vi "A170316-11-Main-large.vi"() -> ()   [LabVIEW 2020]
uses:
  System.Windows.Forms
  Global_Variable/Global.vi
  Database/Global1.vi
  <userlib>/_MGI/Menu Building/MenuItemStatusChange/MGI_MenuItemStatusChange.lvclass
  Libraries/S7/S7.lvlib
panel:
  out "PLC":bool
  out "传感器值":sgl format="%#_5gN"
  out "前序状态字":string
  out "前序状态":bool
  in  "打印条码":bool caption="布尔"
  out "结果显示":string
  in  "质量报警":bool caption="布尔"
  in  "设备缺料":bool caption="布尔"
  in  "设备故障":bool caption="布尔"
  in  "设备离线":bool caption="布尔"
  in  "设备正常":bool caption="布尔"
  in  "菜单":refnum<k24>(container)
  out "检测结果":bool
  in  "批次信息":string[][](table)
  out "提示信息":string
  out "错误":bool
  out "时间字符串":string
  out "日期字符串":string
  out "自动":bool
  out "userStatus":string caption="用户状态"
  out "userName":string caption="用户名"
  out "合格数量":u32
  out "生产数量":u32
  out "追溯码":string
  out "connectionMode":string caption="联机类型"
  out "产品型号":string
  in  "更换产品":refnum<vi>
  # "中间轴装配"
  # "工艺流程"
  # "检测结果："
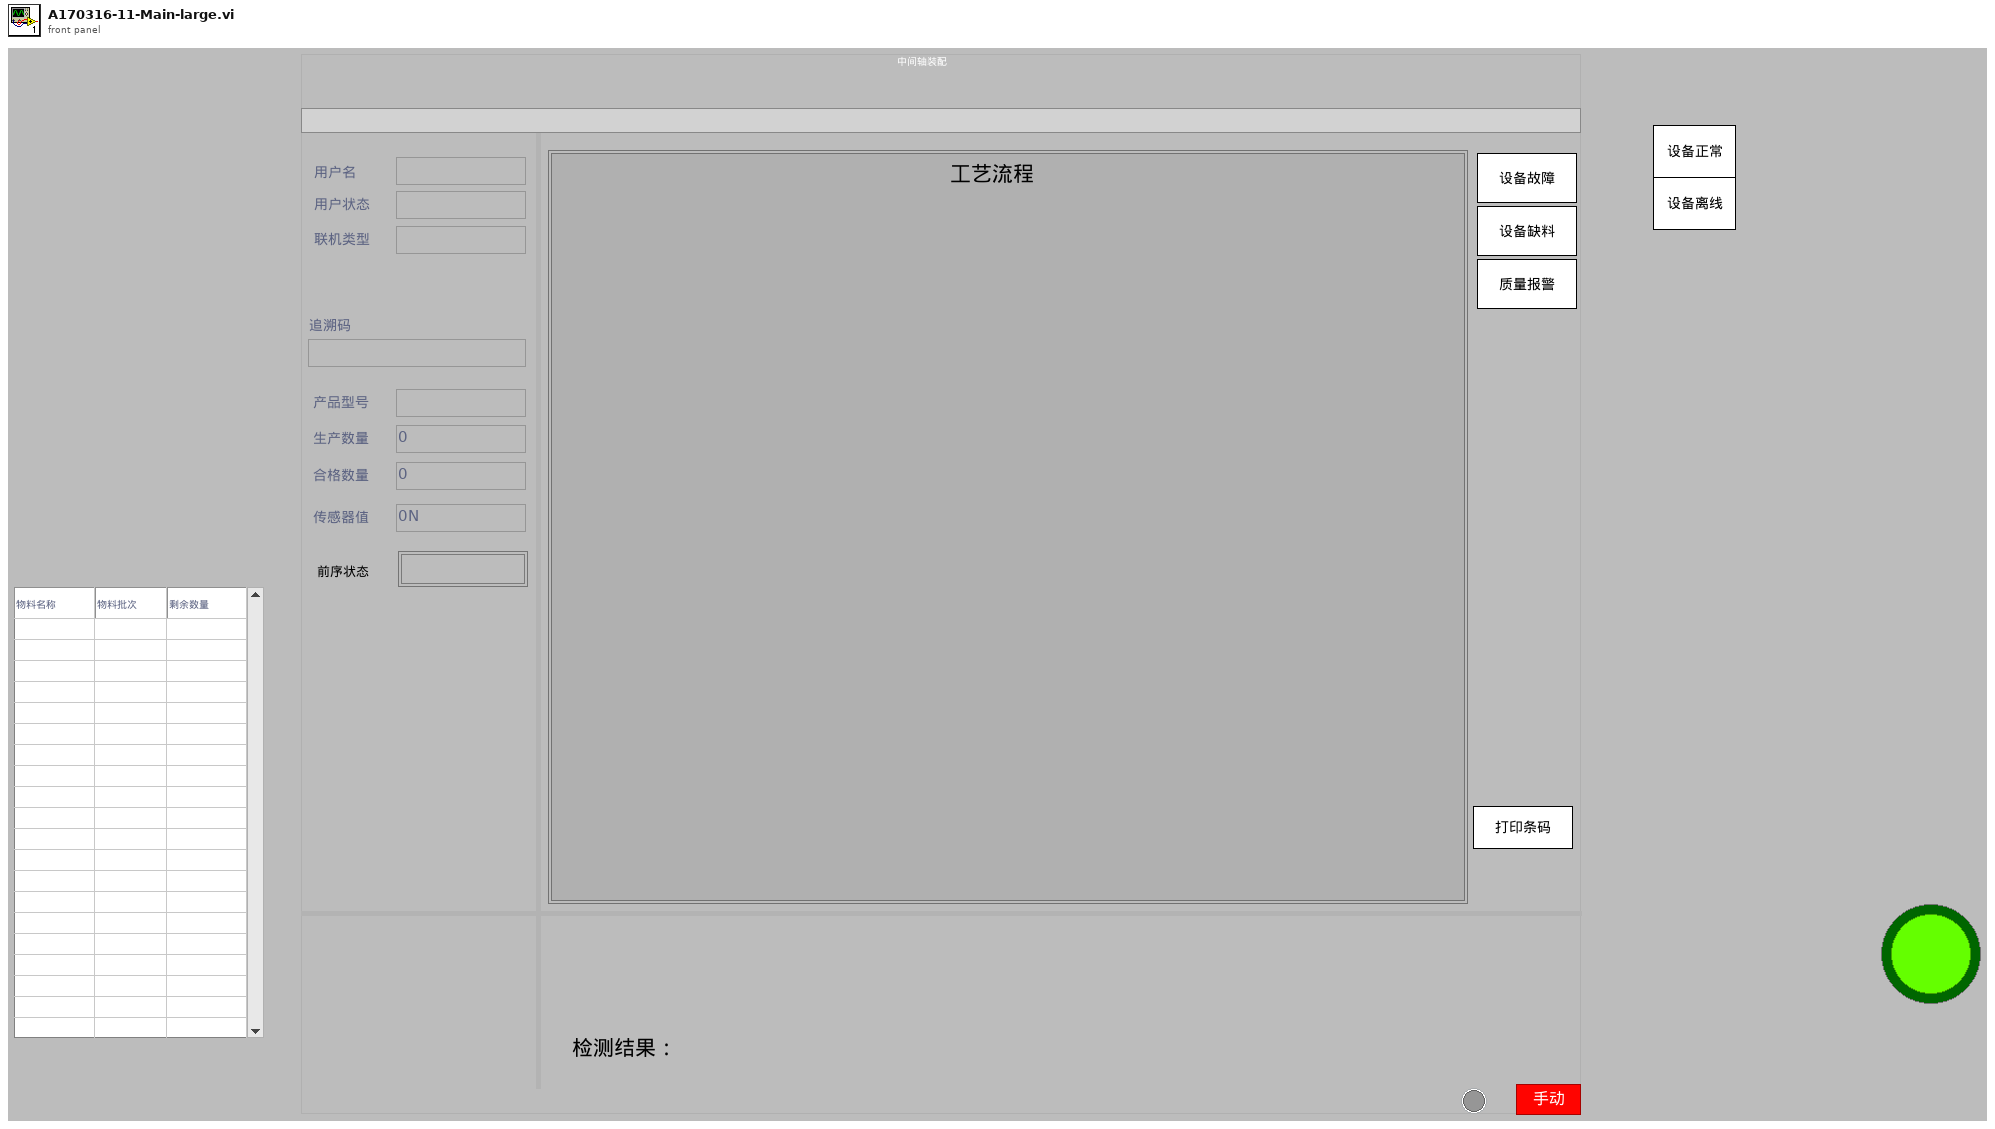
[diagram p1: front panel]
types:
  T1 = typedef "S7.lvlib/Broadcast Events--cluster.ctl" = cluster{"Module Did Init":refnum<user-event>, "Status Updated":refnum<user-event>, "Error Reported":refnum<user-event>, "Module Did Stop":refnum<user-event>, "Update Module Execution Status":refnum<user-event>}
  T2 = enum32{"Invalid", "Standard", "Closed", "Hidden", "Minimized", "Maximized"}
  T3 = enum32{"invalid app kind", "Development System", "Run Time System", "Student Edition", "Embedded LabVIEW", "Evaluation", "Custom"}
  T4 = typedef "S7.lvlib/Read_Data (Reply Payload)--cluster.ctl" = cluster{"读取成功":bool, "数据":u32[], "Read_Data_error":errorcluster}
  T5 = cluster{"Core":cluster{"Current VI Reference":refnum<vi>, "Close Panel on Exit?":bool}, "Your Boolean data":bool, "Your string data":string}
  T6 = cluster{"Current VI Reference":refnum<vi>, "Close Panel on Exit?":bool}
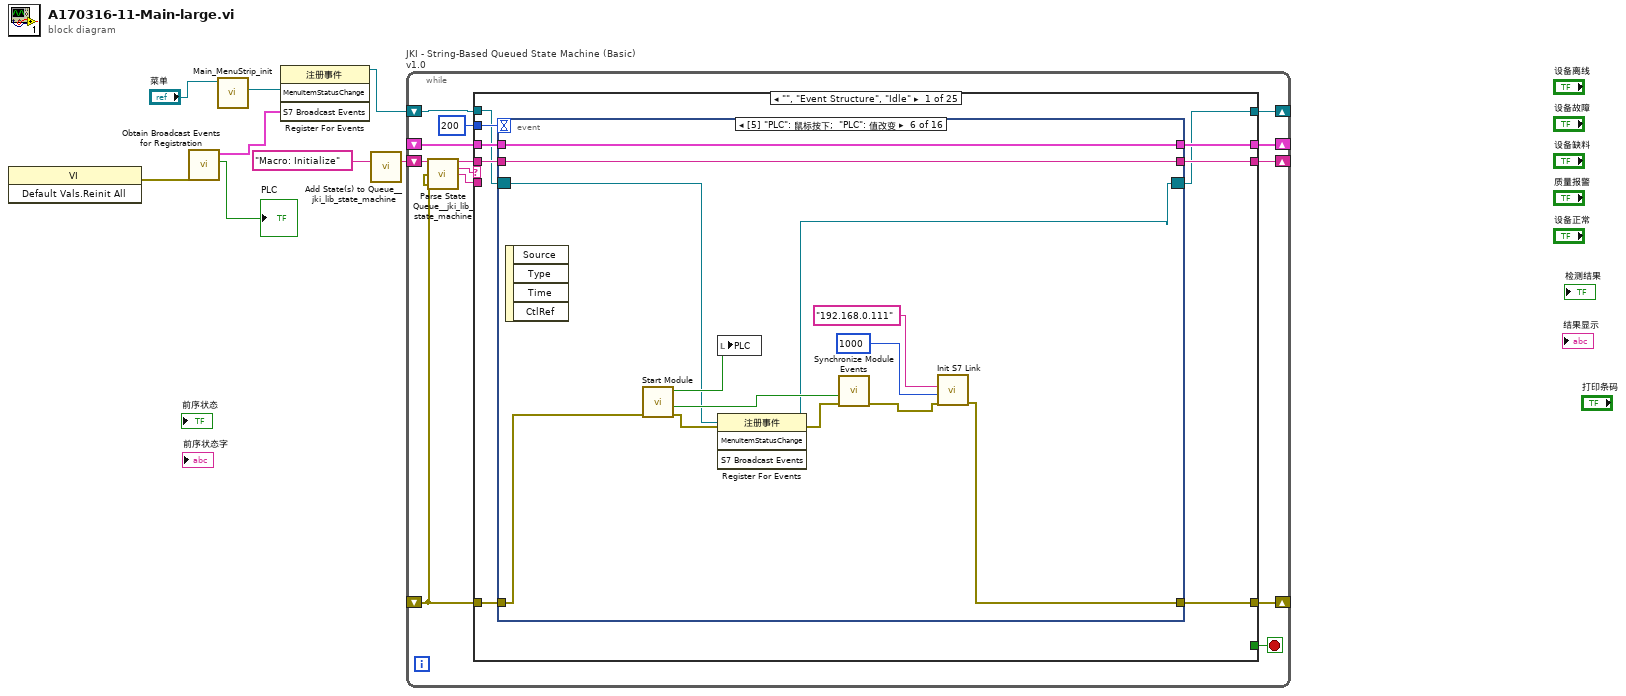
[diagram p0: block diagram]
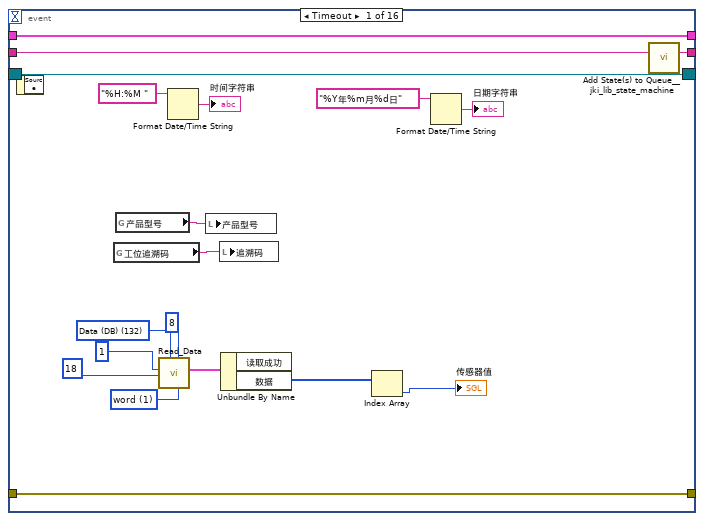
[diagram p2: hidden frame]
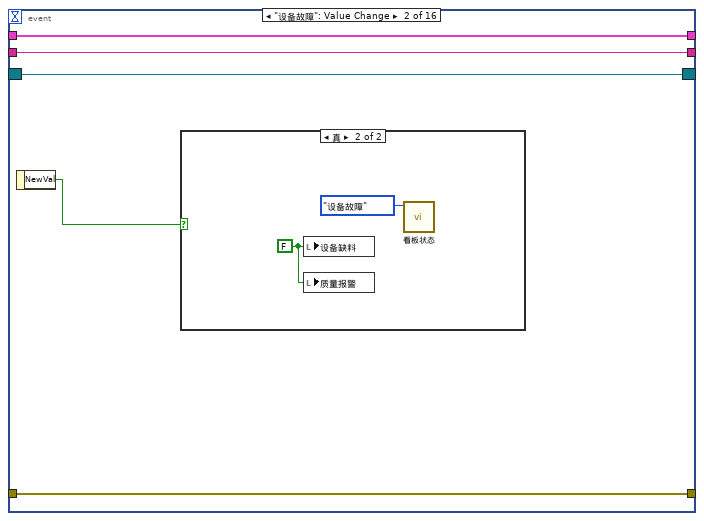
[diagram p3: hidden frame]
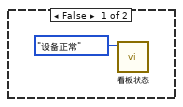
[diagram p4: hidden frame]
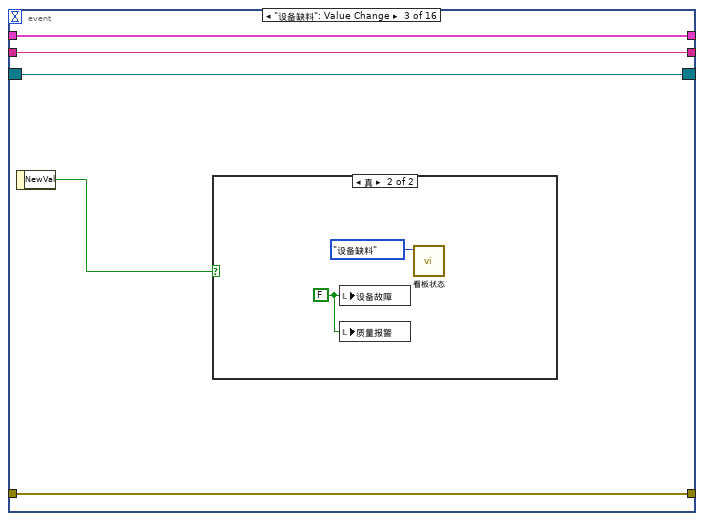
[diagram p5: hidden frame]
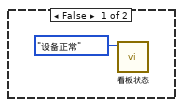
[diagram p6: hidden frame]
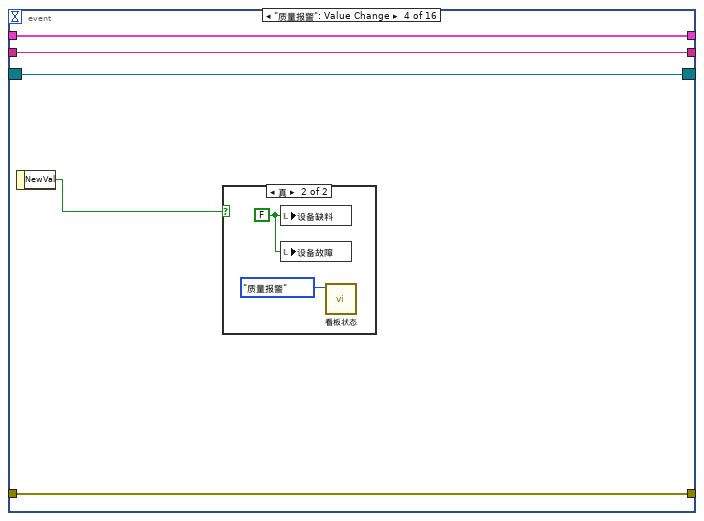
[diagram p7: hidden frame]
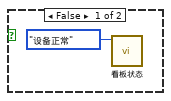
[diagram p8: hidden frame]
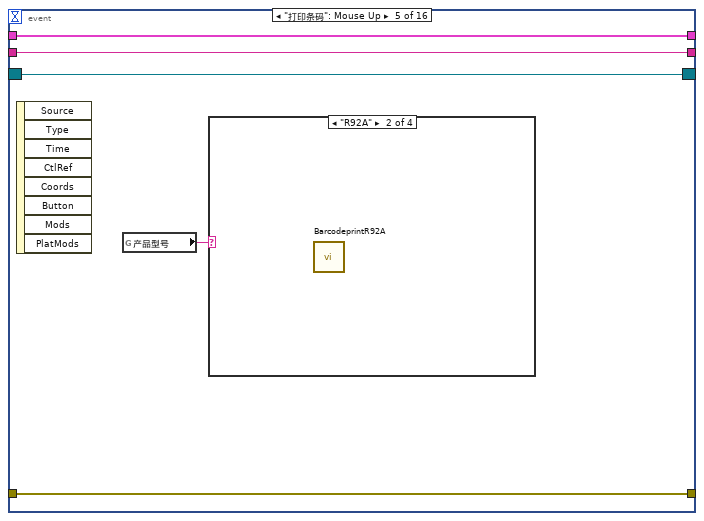
[diagram p9: hidden frame]
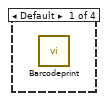
[diagram p10: hidden frame]
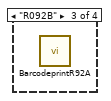
[diagram p11: hidden frame]
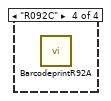
[diagram p12: hidden frame]
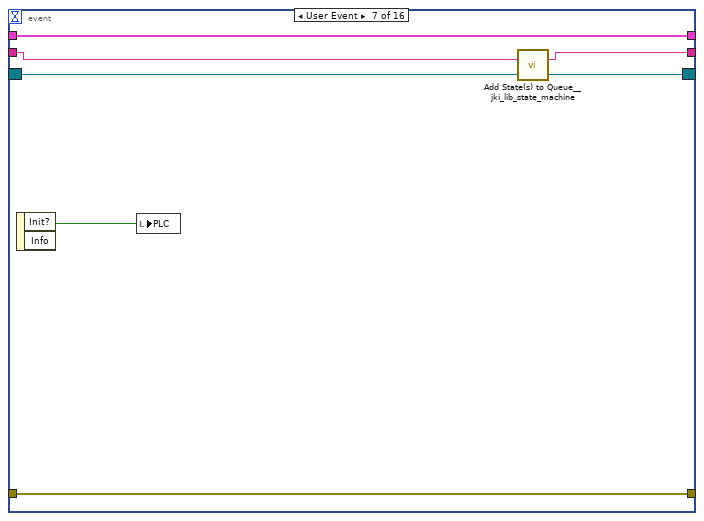
[diagram p13: hidden frame]
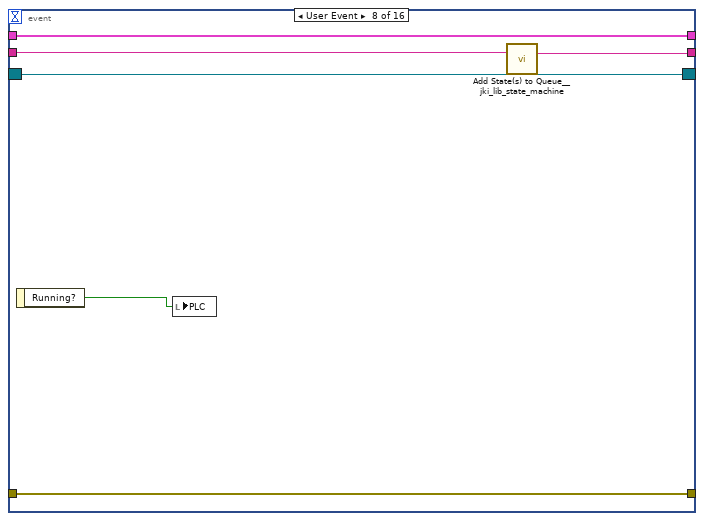
[diagram p14: hidden frame]
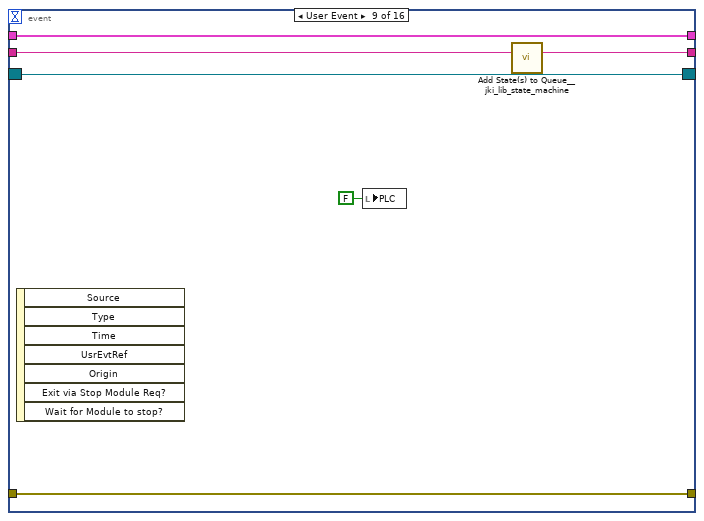
[diagram p15: hidden frame]
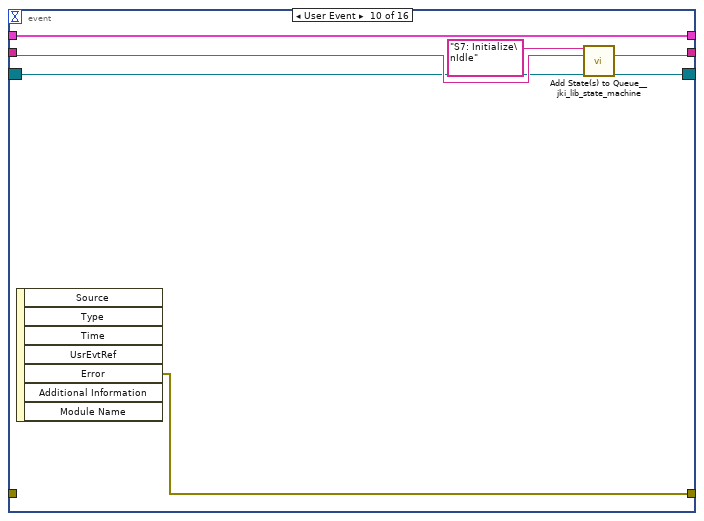
[diagram p16: hidden frame]
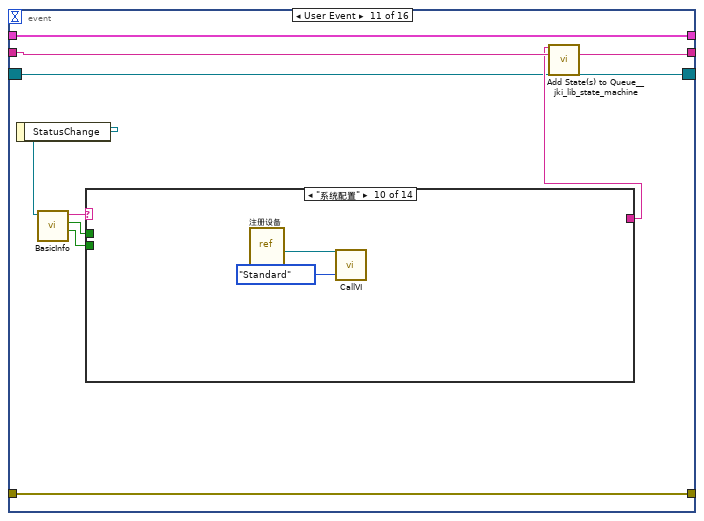
[diagram p17: hidden frame]
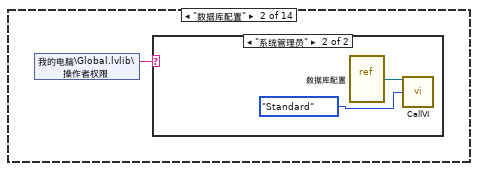
[diagram p19: hidden frame]
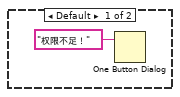
[diagram p20: hidden frame]
diagram:
  n1 = invoke class="VI" method="Default Vals.Reinit All"() -> (error out=w4:errorcluster)  [unwired: 3 in, 2 out]
  n2 = call "Obtain Broadcast Events for Registration.vi"("error in (no error)"=w4) -> ("Already running?"=→"PLC":bool, "S7 Broadcast Events"=w3:T1)  [unwired: 8 in, 1 out]
  n3 = call "Main_MenuStrip_init.vi"("MenuStrip"="菜单") -> ("MenuItemStatusChange"=w5:refnum<user-event>)  [unwired: 9 in, 1 out]
  n4 = register-events(w5, w3) -> (reference out=w2:refnum<event-registration>)  [unwired: 2 in, 1 out]
  n5 = call <vilib>:"Add State(s) to Queue__jki_lib_state_machine.vi"("State(s) in (\"\")"="Macro: Initialize") -> ("States Out"=w8:string)  [unwired: 14 in]
  n6 = while "JKI - String-Based Queued State Machine (Basic) v1.0" {
    shift-right: [w14] -> _
    shift-left: _ -> [w13]
    shift-right: [w17] -> _
    shift-left: _ -> [w11]
    shift-right: [w16] -> _
    shift-left: w8 -> [w18]
    shift-right: [w10] -> _
    shift-left: w2 -> [w9]
    stop <- w15 stop-if-true
    n7 = call <vilib>:"Parse State Queue__jki_lib_state_machine.vi"("State Queue"=w18, "Error In (no error)"=w11) -> ("Remaining States"=w20:string, "Current State"=w21:string, "Arguments"=w19:string)  [unwired: 11 in]
    n8 = case shown="\"\", \"Event Structure\", \"Idle\"" w21 {
      selector: w21 -> [_ _ w261 _ _ _ _ _ _ _ _ _ _ _ _ _ _ _ _ _ _ _ _ _ _]
      tunnel: w20 -> [w30 w259 w265 w283 w289 w294 w298 w305 w311 w315 w316 w323 w327 w331 w335 w347 w351 w390 w401 w427 w432 w445 w449 w453 w457]
      tunnel: w19 -> [_ _ _ _ _ _ _ _ _ _ _ _ _ _ _ _ _ w385 w395 _ _ _ _ _ _]
      tunnel: w13 -> [w28 w256 w263 w274 w286 w292 w295 _ w306 w312 w318 w320 w324 w328 w332 w345 w349 w388 w397 w424 w429 w442 w446 w450 w454]
      tunnel: [w27 w257 w267 w280 errorcluster {"status"=FALSE, "code"=0, "source"=""} ("error out") w291 w296 w302 w307 w313 w319 w321 w325 w329 w333 w342 w348 w386 w398 w425 w430 w443 w447 w451 w455] -> w17
      tunnel: w11 -> [w26 w257 w266 w280 w285 w291 w296 w302 w308 w313 w319 w321 w325 w329 w333 w337 w348 w387 w399 w425 w430 w443 w447 w451 w455]
      tunnel: [w29 w258 w264 w282 w288 w293 w297 w304 w310 w314 w316 w322 w326 w330 w334 w346 w350 w389 w400 w426 w431 w444 w448 w452 w456] -> w16
      tunnel: [_ _ _ _ _ TRUE _ _ _ _ _ _ _ _ _ _ _ _ _ _ _ _ _ _ _] -> w15
      tunnel: [w25 w256 w263 w281 w286 w292 w295 w303 w306 w312 w318 w320 w324 w328 w332 w345 w349 w388 w397 w424 w429 w442 w446 w450 w454] -> w14
      tunnel: 200 ("Timeout") -> [w24 _ _ _ _ _ _ _ _ _ _ _ _ _ _ _ _ _ _ _ _ _ _ _ _]
      tunnel: w9 -> [w23 _ w260 _ _ _ _ _ _ _ _ _ _ _ _ _ _ _ _ _ _ _ _ _ _]
      tunnel: [w22 _ w260 _ _ _ _ _ _ _ _ _ _ _ _ _ _ _ _ _ _ _ _ _ _] -> w10
      frame "", "Event Structure", "Idle" {
        n9 = event shown="[5] \"PLC\": 鼠标按下;  \"PLC\": 值改变" {
          selector: w23 -> [w31 w50 w58 w66 w74 w88 w92 w98 w104 w110 w116 w168 w218 w225 w241 w249]
          dyn-events: [w31 w50 w58 w66 w74 w87 w92 w98 w104 w110 w116 w168 w218 w225 w241 w249] -> w22
          timeout: w24 -> [_ _ _ _ _ _ _ _ _ _ _ _ _ _ _ _]
          tunnel: w30 -> [w49 w53 w61 w69 w76 w85 w95 w102 w107 w111 w120 w171 w222 w229 w248 w252]
          tunnel: [w48 w53 w61 w69 w76 w85 w94 w101 w108 w112 w119 w169 w223 w229 w247 w253] -> w29
          tunnel: w28 -> [w46 w54 w62 w70 w77 w86 w96 w100 w106 w114 w121 w170 w224 w230 w245 w255]
          tunnel: [w47 w52 w60 w68 w75 w79 w93 w99 w105 w115 w117 w172 w221 w228 w246 w254] -> w27
          tunnel: w26 -> [w47 w52 w60 w68 w75 w90 w93 w99 w105 _ w117 w172 w221 w228 w246 w254]
          tunnel: [w46 w54 w62 w70 w77 w86 w96 w100 w106 w114 w121 w170 w224 w230 w245 w255] -> w25
          event Timeout {
            w32 = u16 1 items=["byte", "word", "Dword"] ("数据类型")
            w38 = u8 132 items=["I/O (P)"=128, "Input (I)"=129, "Output (Q)"=130, "Bit Memory (M)"=131, "Data (DB)"=132, "Instance Data (DI)"=133, "Local Data (L)"=134, "Predecessor Local Data (VL)"=135] ("寄存器类型")
            n10 = event-data() -> ()  [unwired: 1 in, 1 out]
            n11 = global read "Global1.vi" "工位追溯码"() -> (w40:string)
            n12 = global read "Global.vi" "产品型号"() -> (w41:string)
            n13 = call "Read_Data.vi"("数据类型"=w32, "读取长度"=u16 8, "寄存器类型"=w38, "起始地址"=u32 18, "DB #"=u16 1) -> ("Reply Payload"=w35:T4)  [unwired: 4 in, 2 out]
            n14 = Format Date/Time String(time format string (%c)="%H:%M ") -> (date/time string=→"时间字符串":string)  [unwired: 2 in]
            n15 = local write "产品型号"(w41) -> ()
            n16 = local write "追溯码"(w40) -> ()
            n17 = Unbundle By Name(w35) -> ("数据"=w34:u32[])  [unwired: 1 out]
            n18 = Index Array(array=w34) -> (element=→"传感器值":u32)  [unwired: 1 in]
            n19 = Format Date/Time String(time format string (%c)="%Y年%m月%d日") -> (date/time string=→"日期字符串":string)  [unwired: 2 in]
            n20 = call <vilib>:"Add State(s) to Queue__jki_lib_state_machine.vi"("State(s) in (\"\")"=w49) -> ("States Out"=w48:string)  [unwired: 14 in]
          }
          event "设备故障": Value Change {
            n21 = event-data() -> ("NewVal"=w51:bool)  [unwired: 1 in]
            n22 = case shown="真" w51 {
              frame False {
                n23 = call "看板状态.vi"("设备状态"=enum16{"设备离线", "设备正常", "设备缺料", "设备故障", "质量报警"}."设备正常") -> ()  [unwired: 10 in, 1 out]
              }
              frame True {
                w56 = FALSE ("质量报警")
                n24 = local write "设备缺料"(w56) -> ()
                n25 = local write "质量报警"(w56) -> ()
                n26 = call "看板状态.vi"("设备状态"=enum16{"设备离线", "设备正常", "设备缺料", "设备故障", "质量报警"}."设备故障") -> ()  [unwired: 10 in, 1 out]
              }
            }
          }
          event "设备缺料": Value Change {
            n27 = event-data() -> ("NewVal"=w59:bool)  [unwired: 1 in]
            n28 = case shown="真" w59 {
              frame False {
                n29 = call "看板状态.vi"("设备状态"=enum16{"设备离线", "设备正常", "设备缺料", "设备故障", "质量报警"}."设备正常") -> ()  [unwired: 10 in, 1 out]
              }
              frame True {
                w64 = FALSE ("质量报警")
                n30 = local write "设备故障"(w64) -> ()
                n31 = local write "质量报警"(w64) -> ()
                n32 = call "看板状态.vi"("设备状态"=enum16{"设备离线", "设备正常", "设备缺料", "设备故障", "质量报警"}."设备缺料") -> ()  [unwired: 10 in, 1 out]
              }
            }
          }
          event "质量报警": Value Change {
            n33 = event-data() -> ("NewVal"=w67:bool)  [unwired: 1 in]
            n34 = case shown="真" w67 {
              frame False {
                n35 = call "看板状态.vi"("设备状态"=enum16{"设备离线", "设备正常", "设备缺料", "设备故障", "质量报警"}."设备正常") -> ()  [unwired: 10 in, 1 out]
              }
              frame True {
                w72 = FALSE ("质量报警")
                n36 = local write "设备缺料"(w72) -> ()
                n37 = local write "设备故障"(w72) -> ()
                n38 = call "看板状态.vi"("设备状态"=enum16{"设备离线", "设备正常", "设备缺料", "设备故障", "质量报警"}."质量报警") -> ()  [unwired: 10 in, 1 out]
              }
            }
          }
          event "打印条码": Mouse Up {
            n39 = event-data() -> ()  [unwired: 1 in, 8 out]
            n40 = global read "Global.vi" "产品型号"() -> (w78:string)
            n41 = case shown="\"R92A\"" w78 {
              frame Default {
                n42 = call "Barcodeprint.vi"() -> ()  [unwired: 12 in]
              }
              frame "R92A" {
                n43 = call "BarcodeprintR92A.vi"() -> ()  [unwired: 12 in]
              }
              frame "R092B" {
                n44 = call "BarcodeprintR92A.vi"() -> ()  [unwired: 12 in]
              }
              frame "R092C" {
                n45 = call "BarcodeprintR92A.vi"() -> ()  [unwired: 12 in]
              }
            }
          }
          event "PLC": Mouse Down; "PLC": Value Change {
            n46 = event-data() -> ()  [unwired: 1 in, 4 out]
            n47 = call "Start Module.vi"("error in (no error)"=w90) -> ("error out"=w80:errorcluster, "Wait for Event Sync?"=w89:bool, "Module Was Already Running?"=w91:bool)  [unwired: 7 in, 1 out]
            n48 = local write "PLC"(w91) -> ()
            n49 = register-events(reference=w88, error in=w80) -> (reference out=w87:refnum<event-registration>, error out=w81:errorcluster)  [unwired: 2 in]
            n50 = call "Synchronize Module Events.vi"("error in (no error)"=w81, "Wait for Event Sync?"=w89) -> ("error out"=w82:errorcluster)  [unwired: 9 in]
            n51 = call "Init S7 Link.vi"("error in (no error)"=w82, "超时"=1000, "IP"="192.168.0.111" ("Origin")) -> ("error out"=w79:errorcluster)  [unwired: 8 in]
          }
          event User Event {
            n52 = event-data() -> ("Init?"=w97:bool)  [unwired: 1 in, 1 out]
            n53 = local write "PLC"(w97) -> ()
            n54 = call <vilib>:"Add State(s) to Queue__jki_lib_state_machine.vi"("State(s) in (\"\")"=w95) -> ("States Out"=w94:string)  [unwired: 14 in]
          }
          event User Event {
            n55 = event-data() -> ("Running?"=w103:bool)  [unwired: 1 in]
            n56 = local write "PLC"(w103) -> ()
            n57 = call <vilib>:"Add State(s) to Queue__jki_lib_state_machine.vi"("State(s) in (\"\")"=w102) -> ("States Out"=w101:string)  [unwired: 14 in]
          }
          event User Event {
            n58 = event-data() -> ()  [unwired: 1 in, 7 out]
            n59 = local write "PLC"(FALSE ("PLC")) -> ()
            n60 = call <vilib>:"Add State(s) to Queue__jki_lib_state_machine.vi"("State(s) in (\"\")"=w107) -> ("States Out"=w108:string)  [unwired: 14 in]
          }
          event User Event {
            n61 = event-data() -> ("Error"=w115:errorcluster)  [unwired: 1 in, 6 out]
            n62 = call <vilib>:"Add State(s) to Queue__jki_lib_state_machine.vi"("State(s) in Front (\"\")"="S7: Initialize\nIdle" ("State(s) in Front (\"\")"), "State(s) in (\"\")"=w111) -> ("States Out"=w112:string)  [unwired: 13 in]
          }
          event User Event {
            n63 = event-data() -> ("StatusChange"=w122:refnum<class "MGI_MenuItemStatusChange.lvclass">)  [unwired: 1 in]
            n64 = call <userlib>:"BasicInfo.vi"("MGI_MenuItemStatusChange in"=w122) -> ("Enabled?"=w125:bool, "Checked?"=w124:bool, "Tag"=w123:string)  [unwired: 7 in, 1 out]
            n65 = case shown="\"系统配置\"" w123 {
              tunnel: w124 -> [_ _ _ _ _ _ _ _ _ _ _ _ _ _]
              tunnel: w125 -> [_ _ _ _ _ _ _ _ _ _ _ _ _ _]
              tunnel: [_ _ "Macro: Exit" _ _ _ _ _ _ _ _ _ _ _] -> w118
              frame Default {
              }
              frame "数据库配置" {
                n66 = shared-variable "我的电脑\\Global.lvlib\\操作者权限"() -> (w126:string)  [unwired: 1 in, 1 out]
                n67 = case shown="\"系统管理员\"" w126 {
                  frame Default {
                    n68 = One Button Dialog(message="权限不足！" ("消息")) -> ()  [unwired: 1 in, 1 out]
                  }
                  frame "系统管理员" {
                    n69 = vi-ref "数据库配置.vi"() -> (w129:refnum<vi>)
                    n70 = call "CallVI.vi"("VI引用"=w129, "状态"=T2."Standard") -> ()  [unwired: 11 in, 3 out]
                  }
                }
              }
              frame "退出" {
              }
              frame "手动控制" {
                n71 = shared-variable "我的电脑\\Global.lvlib\\操作者权限"() -> (w131:string)  [unwired: 1 in, 1 out]
                n72 = case shown="\"班组长\", \"系统管理员\"" w131 {
                  frame Default {
                    n73 = One Button Dialog(message="权限不足！" ("消息")) -> ()  [unwired: 1 in, 1 out]
                  }
                  frame "班组长", "系统管理员" {
                    n74 = vi-ref "A170316-11_IO.vi"() -> (w134:refnum<vi>)
                    n75 = call "CallVI.vi"("VI引用"=w134, "状态"=T2."Standard") -> ()  [unwired: 11 in, 3 out]
                  }
                }
              }
              frame "产品管理" {
                n76 = vi-ref "A170316-11_config.vi"() -> (w136:refnum<vi>)
                n77 = call "CallVI.vi"("VI引用"=w136, "状态"=T2."Standard") -> ()  [unwired: 11 in, 3 out]
              }
              frame "用户管理" {
                n78 = shared-variable "我的电脑\\Global.lvlib\\操作者权限"() -> (w137:string)  [unwired: 1 in, 1 out]
                n79 = case shown="\"系统管理员\"" w137 {
                  frame Default {
                    n80 = One Button Dialog(message="权限不足！" ("消息")) -> ()  [unwired: 1 in, 1 out]
                  }
                  frame "系统管理员" {
                    n81 = vi-ref "User_manager.vi"() -> (w140:refnum<vi>)
                    n82 = call "CallVI.vi"("VI引用"=w140, "状态"=T2."Standard") -> ()  [unwired: 11 in, 3 out]
                  }
                }
              }
              frame "编码规则" {
                n83 = shared-variable "我的电脑\\Global.lvlib\\操作者权限"() -> (w141:string)  [unwired: 1 in, 1 out]
                n84 = case shown="\"班组长\", \"工艺管理员\", \"系统管理员\"" w141 {
                  frame Default {
                    n85 = One Button Dialog(message="权限不足！" ("消息")) -> ()  [unwired: 1 in, 1 out]
                  }
                  frame "班组长", "工艺管理员", "系统管理员" {
                    n86 = vi-ref "编码规则设置.vi"() -> (w144:refnum<vi>)
                    n87 = call "CallVI.vi"("VI引用"=w144, "状态"=T2."Standard") -> ()  [unwired: 11 in, 3 out]
                  }
                }
              }
              frame "易损件管理" {
                n88 = vi-ref "易损件管理.vi"() -> (w146:refnum<vi>)
                n89 = call "CallVI.vi"("VI引用"=w146, "状态"=T2."Standard") -> ()  [unwired: 11 in, 3 out]
              }
              frame "物料批次管理" {
                n90 = vi-ref "批次管理.vi"() -> (w148:refnum<vi>)
                n91 = call "CallVI.vi"("VI引用"=w148, "状态"=T2."Standard") -> ()  [unwired: 11 in, 3 out]
              }
              frame "系统配置" {
                n92 = vi-ref "注册设备.vi"() -> (w150:refnum<vi>)
                n93 = call "CallVI.vi"("VI引用"=w150, "状态"=T2."Standard") -> ()  [unwired: 11 in, 3 out]
              }
              frame "报表" {
                n94 = call "文件对话框2"("start path"=path "D:/report", "prompt"="打开报表", "pattern (all files)"="*.doc;*.docx", "pattern label"="Word 文档") -> ("selected path"=w151:path, "error out"=w152:errorcluster)  [unwired: 8 in, 2 out]
                n95 = case shown="无错误" w152 {
                  selector: w152 -> [w158 w160]
                  tunnel: w151 -> [w159 _]
                  frame No Error {
                    w157 = 1 items=["Normal", "Maximize", "Minimize"] ("cpubbs_WindowState")
                    n96 = call "Open_Word.vi"("File Path"=w159, "cpubbs_WindowState"=w157, "错误输入（无错误）"=w158) -> ()  [unwired: 12 in, 1 out]
                  }
                  frame Error {
                    n97 = call <vilib>:"Clear Errors.vi"("error in (no error)"=w160) -> ()  [unwired: 5 in, 2 out]
                  }
                }
              }
              frame "报警信息" {
                n98 = vi-ref "报警信息.vi"() -> (w162:refnum<vi>)
                n99 = call "CallVI.vi"("VI引用"=w162, "状态"=T2."Standard") -> ()  [unwired: 11 in, 3 out]
              }
              frame "关于" {
                n100 = vi-ref "About.vi"() -> (w164:refnum<vi>)
                n101 = call "CallVI.vi"("VI引用"=w164, "状态"=T2."Standard") -> ()  [unwired: 11 in, 3 out]
              }
              frame "操作演示" {
                n102 = call <vilib>:"Application Directory.vi"() -> ("Application Directory"=w167:path)
                n103 = Build Path(base path=w167, name or relative path="操作演示" ("名称或相对路径")) -> (appended path=w166:path)
                n104 = call "自动播放ppt.vi"("路径"=w166) -> ()  [unwired: 10 in, 1 out]
              }
            }
            n105 = call <vilib>:"Add State(s) to Queue__jki_lib_state_machine.vi"("State(s) in Front (\"\")"=w118, "State(s) in (\"\")"=w120) -> ("States Out"=w119:string)  [unwired: 13 in]
          }
          event Menu Selection (User) {
            n106 = event-data() -> ("ItemTag"=w173:string)  [unwired: 1 in, 6 out]
            n107 = case shown="\"产品管理\"" w173 {
              frame "假", Default {
              }
              frame "数据库配置" {
                n108 = shared-variable "我的电脑\\Global.lvlib\\操作者权限"() -> (w174:string)  [unwired: 1 in, 1 out]
                n109 = case shown="\"系统管理员\"" w174 {
                  frame Default {
                    n110 = One Button Dialog(message="权限不足！" ("消息")) -> ()  [unwired: 1 in, 1 out]
                  }
                  frame "系统管理员" {
                    n111 = vi-ref "数据库配置.vi"() -> (w177:refnum<vi>)
                    n112 = call "CallVI.vi"("VI引用"=w177, "状态"=T2."Standard") -> ()  [unwired: 11 in, 3 out]
                  }
                }
              }
              frame "退出" {
                n113 = Quit LabVIEW() -> ()  [unwired: 1 in]
              }
              frame "手动控制" {
                n114 = shared-variable "我的电脑\\Global.lvlib\\操作者权限"() -> (w178:string)  [unwired: 1 in, 1 out]
                n115 = case shown="\"班组长\", \"系统管理员\"" w178 {
                  frame Default {
                    n116 = One Button Dialog(message="权限不足！" ("消息")) -> ()  [unwired: 1 in, 1 out]
                  }
                  frame "班组长", "系统管理员" {
                    n117 = vi-ref "A170316-11_IO.vi"() -> (w181:refnum<vi>)
                    n118 = call "CallVI.vi"("VI引用"=w181, "状态"=T2."Standard") -> ()  [unwired: 11 in, 3 out]
                  }
                }
              }
              frame "半自动控制" {
                n119 = disable-structure shown="启用" {
                  frame Disabled {
                    n120 = shared-variable "我的电脑\\Global.lvlib\\操作者权限"() -> (w182:string)  [unwired: 1 in, 1 out]
                    n121 = case shown="\"班组长\", \"系统管理员\"" w182 {
                      frame Default {
                        n122 = One Button Dialog(message="权限不足！" ("消息")) -> ()  [unwired: 1 in, 1 out]
                      }
                      frame "班组长", "系统管理员" {
                        n123 = call "CallVI.vi"("VI引用"=refnum<vi> refnum, "状态"=T2."Maximized") -> ()  [unwired: 11 in, 3 out]
                      }
                    }
                  }
                  frame Enabled {
                    n124 = One Button Dialog(message="当前设备不具备半自动功能！" ("消息")) -> ()  [unwired: 1 in, 1 out]
                  }
                }
              }
              frame "产品管理" {
                n125 = vi-ref "A170316-11_config.vi"() -> (w188:refnum<vi>)
                n126 = call "CallVI.vi"("VI引用"=w188, "状态"=T2."Standard") -> ()  [unwired: 11 in, 3 out]
              }
              frame "系统配置" {
              }
              frame "用户管理" {
                n127 = shared-variable "我的电脑\\Global.lvlib\\操作者权限"() -> (w189:string)  [unwired: 1 in, 1 out]
                n128 = case shown="\"系统管理员\"" w189 {
                  frame Default {
                    n129 = One Button Dialog(message="权限不足！" ("消息")) -> ()  [unwired: 1 in, 1 out]
                  }
                  frame "系统管理员" {
                    n130 = vi-ref "User_manager.vi"() -> (w192:refnum<vi>)
                    n131 = call "CallVI.vi"("VI引用"=w192, "状态"=T2."Standard") -> ()  [unwired: 11 in, 3 out]
                  }
                }
              }
              frame "编码规则" {
                n132 = shared-variable "我的电脑\\Global.lvlib\\操作者权限"() -> (w193:string)  [unwired: 1 in, 1 out]
                n133 = case shown="\"班组长\", \"工艺管理员\", \"系统管理员\"" w193 {
                  frame Default {
                    n134 = One Button Dialog(message="权限不足！" ("消息")) -> ()  [unwired: 1 in, 1 out]
                  }
                  frame "班组长", "工艺管理员", "系统管理员" {
                    n135 = vi-ref "编码规则设置.vi"() -> (w196:refnum<vi>)
                    n136 = call "CallVI.vi"("VI引用"=w196, "状态"=T2."Standard") -> ()  [unwired: 11 in, 3 out]
                  }
                }
              }
              frame "易损件管理" {
                n137 = vi-ref "易损件管理.vi"() -> (w198:refnum<vi>)
                n138 = call "CallVI.vi"("VI引用"=w198, "状态"=T2."Standard") -> ()  [unwired: 11 in, 3 out]
              }
              frame "物料批次管理" {
                n139 = vi-ref "批次管理.vi"() -> (w200:refnum<vi>)
                n140 = call "CallVI.vi"("VI引用"=w200, "状态"=T2."Standard") -> ()  [unwired: 11 in, 3 out]
              }
              frame "打开报表" {
                n141 = call "文件对话框"("start path"=path "D:/report", "prompt"="打开报表", "pattern (all files)"="*.doc;*.docx", "pattern label"="Word 文档") -> ("selected path"=w201:path, "error out"=w202:errorcluster)  [unwired: 8 in, 2 out]
                n142 = case shown="无错误" w202 {
                  selector: w202 -> [w208 w210]
                  tunnel: w201 -> [w209 _]
                  frame No Error {
                    w207 = 1 items=["Normal", "Maximize", "Minimize"] ("cpubbs_WindowState")
                    n143 = call "Open_Word.vi"("File Path"=w209, "cpubbs_WindowState"=w207, "错误输入（无错误）"=w208) -> ()  [unwired: 12 in, 1 out]
                  }
                  frame Error {
                    n144 = call <vilib>:"Clear Errors.vi"("error in (no error)"=w210) -> ()  [unwired: 5 in, 2 out]
                  }
                }
              }
              frame "报警信息" {
                n145 = vi-ref "报警信息.vi"() -> (w212:refnum<vi>)
                n146 = call "CallVI.vi"("VI引用"=w212, "状态"=T2."Standard") -> ()  [unwired: 11 in, 3 out]
              }
              frame "关于" {
                n147 = vi-ref "About.vi"() -> (w214:refnum<vi>)
                n148 = call "CallVI.vi"("VI引用"=w214, "状态"=T2."Standard") -> ()  [unwired: 11 in, 3 out]
              }
              frame "操作演示" {
                n149 = call <vilib>:"Application Directory.vi"() -> ("Application Directory"=w217:path)
                n150 = Build Path(base path=w217, name or relative path="操作演示" ("名称或相对路径")) -> (appended path=w216:path)
                n151 = call "自动播放ppt.vi"("路径"=w216) -> ()  [unwired: 10 in, 1 out]
              }
            }
            n152 = call <vilib>:"Add State(s) to Queue__jki_lib_state_machine.vi"("State(s) in (\"\")"=w171) -> ("States Out"=w169:string)  [unwired: 14 in]
          }
          event "错误": Mouse Down {
            n153 = event-data() -> ()  [unwired: 1 in, 8 out]
            n154 = vi-ref "报警信息.vi"() -> (w220:refnum<vi>)
            n155 = call "CallVI.vi"("VI引用"=w220, "状态"=T2."Standard") -> ()  [unwired: 11 in, 3 out]
            n156 = call <vilib>:"Add State(s) to Queue__jki_lib_state_machine.vi"("State(s) in (\"\")"=w222) -> ("States Out"=w223:string)  [unwired: 14 in]
          }
          event "自动": Mouse Down {
            n157 = event-data() -> ("CtlRef"=w227:refnum<vi>)  [unwired: 1 in, 7 out]
            n158 = property class="Bool (严格)"(reference=w227) -> ("Value"=w226:bool)  [unwired: 1 in, 2 out]
            n159 = case shown="真" w226 {
              frame False {
                n160 = shared-variable "我的电脑\\A17031611.lvlib\\设备状态"() -> (w231:i16)  [unwired: 1 in, 1 out]
                n161 = case shown="5" w231 {
                  frame 0, Default {
                    n162 = call "浮动通知.vi"("通知内容"="请复位！") -> ()  [unwired: 11 in]
                  }
                  frame 5 {
                    n163 = vi-ref "A170316-11_Auto.vi"() -> (w235:refnum<vi>)
                    n164 = invoke class="VI" method="Ctrl Val.Set"(reference=w235, "Control Name"="STEP" ("控件名"), "Value"="初始化" ("控件名")) -> ()  [unwired: 2 in, 5 out]
                  }
                }
              }
              frame True {
                n165 = Two Button Dialog(message="自动程序运行中，\n是否切换为手动？" ("消息")) -> (T button?=w236:bool)  [unwired: 2 in]
                n166 = case shown="真" w236 {
                  frame False {
                  }
                  frame True {
                    n167 = vi-ref "A170316-11_Auto.vi"() -> (w240:refnum<vi>)
                    n168 = invoke class="VI" method="Ctrl Val.Set"(reference=w240, "Control Name"="STEP" ("控件名"), "Value"="手动" ("控件名")) -> ()  [unwired: 2 in, 5 out]
                  }
                }
              }
            }
          }
          event Panel Close? {
            n169 = event-data() -> ()  [unwired: 1 in, 1 out]
            n170 = global write "Global.vi" "程序关闭"(TRUE ("程序关闭")) -> ()
            n171 = event-data("Discard?"=TRUE) -> ()  [unwired: 1 in, 1 out]
            n172 = call <vilib>:"Add State(s) to Queue__jki_lib_state_machine.vi"("State(s) in Front (\"\")"="Macro: Exit", "State(s) in (\"\")"=w248) -> ("States Out"=w247:string)  [unwired: 13 in]
          }
          event "更换产品": Value Change {
            n173 = event-data() -> ("NewVal"=w251:refnum<vi>)  [unwired: 1 in, 5 out]
            n174 = control-ref of="子面板"() -> (w250:refnum<vi>)
            n175 = call "Call_SubPanal.vi"("VI引用句柄"=w251, "SubPnl引用句柄"=w250) -> ()  [unwired: 9 in, 1 out]
            n176 = call <vilib>:"Add State(s) to Queue__jki_lib_state_machine.vi"("State(s) in (\"\")"=w252) -> ("States Out"=w253:string)  [unwired: 14 in]
          }
        }
      }
      frame "---------- Core ----------" {
        n177 = call <vilib>:"Add State(s) to Queue__jki_lib_state_machine.vi"("State(s) in (\"\")"=w259) -> ("States Out"=w258:string)  [unwired: 14 in]
      }
      frame Default {
        w270 = 42 items=["No error", "Argument error", "Memory is full", "Out of zone", "End of file", "File already open", "Generic file I/O error", "File not found", "File permission error", "Disk is full", "Duplicate path", "Too many files open", "System feature not enabled", "Resource file not found", "Cannot add resource", "Resource not found", "Image not found", "Image memory error", "Pen does not exist", "Config type invalid", "Config token not found", "Config parse error", "Config memory error", "Bad external code format", "Bad external code offset", "External code not present", "Null window", "Destroy window error", "Null menu", "Print aborted", "Bad print record", "Print driver error", "Windows error during printing", "Memory error during printing", "Print dialog error", "Generic print error", "Invalid device refnum", "Device not found", "Device parameter error", "Device unit error", "Cannot open device", "Device call aborted", "Generic error", "Cancelled by user", "Object ID too low", "Object ID too high", "Object not in heap", "Unknown heap", "Unknown object (invalid DefProc)", "Unknown object (DefProc not in table)", "Message out of range", "Invalid (null) method", "Unknown message", "Manager call not supported", "Bad address", "Network operation in progress", "Network operation timed out", "Connection is busy", "Network attribute not supported", "Network error", "Address in use", "System out of memory", "Connection aborted", "Connection refused", "Not connected", "Already connected", "Connection closed", "Initialization error (interapplication manager)", "Bad occurrence", "Wait on unbound occurrence handler", "Occurrence queue overflow", "Datalog type conflict", "Unused", "Unrecognized type (interapplication manager)", "Memory corrupt", "Failed to make temporary DLL", "Old CIN version", "Drag socket not found", "Failed to load drop-object", "Failed to register OLE object", "Failed to release OLE object", "Format specifier type mismatch", "Unknown format specifier", "Too few format specifiers", "Too many format specifiers", "Scan failed", "Newer CIN version", "Error converting to variant", "Runtime menu error", "Password tampered", "Variant attribute not found", "Incompatible variant data type", "Event data is not available", "Event Store is not present", "Occurrence is not found", "Event Queue is not created", "Event info is not available", "Refnum passed is NULL", "Error retrieving Class GUID", "Error retrieving CoClass GUID", "Error retrieving TypeLib GUID.", "Bad built application magic bytes.", "Specific driver is different from the specific driver associated with the Logical Name.", "There is no session opened to the class driver.", "Max Error", "MAX - Error with config objects", "MAX - Error loading configuration", "MAX - Group not supported"]
        # "Current State"
        n178 = Format Into String(format string="Software Exception: Unhandled State \"%s\"." ("message"), error in=w266, w261) -> (resulting string=w269:string, error out=w268:errorcluster)  [unwired: 1 in]
        n179 = call <vilib>:"Error Cluster From Error Code.vi"("show call chain? (False)"=TRUE, "error in (no error)"=w268, "error message (\"\")"=w269, "error code (0)"=w270) -> ("error out"=w267:errorcluster)  [unwired: 5 in]
        n180 = call <vilib>:"Add State(s) to Queue__jki_lib_state_machine.vi"("State(s) in (\"\")"=w265) -> ("States Out"=w264:string)  [unwired: 14 in]
      }
      frame "Initialize Core Data" {
        # "originally closed?"
        # "exe?"
        n181 = property class="VI"() -> ("Front Panel.Open"=w279:bool)  [unwired: 2 in, 2 out]
        n182 = property class="App"() -> ("App.Kind"=w278:T3)  [unwired: 2 in, 2 out]
        n183 = control-ref of="Current VI Reference"() -> (w272:refnum<vi>)
        n184 = Not(x=w279) -> (.not. x?=w276:bool)
        n185 = Equal?(x=w278, y=T3."Run Time System" ("Application:Kind")) -> (x = y?=w275:bool)
        n186 = Or(x=w276, y=w275) -> (x .or. y?=w273:bool)
        n187 = Bundle By Name(cluster=w274, "Core.Current VI Reference"=w272, "Core.Close Panel on Exit?"=w273) -> (w281:T5)
        n188 = call <vilib>:"Add State(s) to Queue__jki_lib_state_machine.vi"("State(s) in (\"\")"=w283) -> ("States Out"=w282:string)  [unwired: 14 in]
      }
      frame "Error Handler" {
        n189 = call <vilib>:"General Error Handler.vi"("error in (no error)"=w285) -> ()  [unwired: 10 in, 5 out]
        n190 = call <vilib>:"Add State(s) to Queue__jki_lib_state_machine.vi"("State(s) in Front (\"\")"="/* Post Error States", "State(s) in (\"\")"=w289) -> ("States Out"=w288:string)  [unwired: 13 in]
      }
      frame "Exit" {
        n191 = call <vilib>:"Add State(s) to Queue__jki_lib_state_machine.vi"("State(s) in (\"\")"=w294) -> ("States Out"=w293:string)  [unwired: 14 in]
      }
      frame "---------- Data ----------" {
        n192 = call <vilib>:"Add State(s) to Queue__jki_lib_state_machine.vi"("State(s) in (\"\")"=w298) -> ("States Out"=w297:string)  [unwired: 14 in]
      }
      frame "Data: Initialize" {
        w299 = T6 {"Current VI Reference"=refnum, "Close Panel on Exit?"=FALSE}  # Core
        w301 = TRUE  # Your Boolean data
        w300 = ""  # Your string data
        n193 = Bundle("Core"=w299, "Your Boolean data"=w301, "Your string data"=w300) -> (w303:T5)  [unwired: 1 in]
        n194 = call <vilib>:"Add State(s) to Queue__jki_lib_state_machine.vi"("State(s) in (\"\")"=w305) -> ("States Out"=w304:string)  [unwired: 14 in]
      }
      frame "Data: Cleanup" {
        n195 = Unbundle By Name(w306) -> ("Core.Current VI Reference"=w309:refnum<vi>)
        n196 = Close Reference(reference=w309, error in (no error)=w308) -> (error out=w307:errorcluster)
        n197 = call <vilib>:"Add State(s) to Queue__jki_lib_state_machine.vi"("State(s) in (\"\")"=w311) -> ("States Out"=w310:string)  [unwired: 14 in]
      }
      frame "----------Libraries ----------" {
        n198 = call <vilib>:"Add State(s) to Queue__jki_lib_state_machine.vi"("State(s) in (\"\")"=w315) -> ("States Out"=w314:string)  [unwired: 14 in]
      }
      frame "S7: Initialize" {
        n199 = property on="PLC" class="Bool (严格)"("Val(Sgnl)"=FALSE ("值(信号)")) -> ()  [unwired: 2 in, 2 out]
      }
      frame "S7: Stop" {
        n200 = call <vilib>:"Add State(s) to Queue__jki_lib_state_machine.vi"("State(s) in (\"\")"=w323) -> ("States Out"=w322:string)  [unwired: 14 in]
      }
      frame "CAN: Start" {
        n201 = call <vilib>:"Add State(s) to Queue__jki_lib_state_machine.vi"("State(s) in (\"\")"=w327) -> ("States Out"=w326:string)  [unwired: 14 in]
      }
      frame "CAN: Stop" {
        n202 = call <vilib>:"Add State(s) to Queue__jki_lib_state_machine.vi"("State(s) in (\"\")"=w331) -> ("States Out"=w330:string)  [unwired: 14 in]
      }
      frame "---------- UI ----------" {
        # "Do not put any code in this frame.\n(It is a separator no-op. You can make a copy of this frame to create a new UI frame)"
        n203 = call <vilib>:"Add State(s) to Queue__jki_lib_state_machine.vi"("State(s) in (\"\")"=w335) -> ("States Out"=w334:string)  [unwired: 14 in]
      }
      frame "UI: Initialize" {
        n204 = vi-ref "A170316-11_Auto.vi"() -> (w336:refnum<vi>)
        n205 = invoke on="子面板" class="SubPnl" method="Insert VI"(error in=w337, "VI Ref"=w336) -> (error out=w338:errorcluster)  [unwired: 2 in, 3 out]
        n206 = invoke class="VI" method="Run VI"(reference=w336, error in=w338, "Wait until done"=FALSE ("结束前等待"), "Auto Dispose Ref"=TRUE ("自动销毁引用")) -> (error out=w341:errorcluster)  [unwired: 1 in, 4 out]
        n207 = call "窗口自动调整.vi"("error in (no error)"=w341, "max？"=TRUE, "border spacing (2 px)"=0) -> ("error out"=w342:errorcluster)  [unwired: 3 in, 1 out]
        n208 = call <vilib>:"Add State(s) to Queue__jki_lib_state_machine.vi"("State(s) in (\"\")"=w347) -> ("States Out"=w346:string)  [unwired: 14 in]
      }
      frame "UI: Init" {
        n209 = stacked-sequence {
          frame #0 {
            w354 = u32 0 ("合格数量")
            n210 = shared-variable "我的电脑\\Global.lvlib\\联机模式"() -> (w357:i16)  [unwired: 1 in, 1 out]
            n211 = control-ref of="前序状态"() -> (w353:refnum<vi>)
            n212 = control-ref of="前序状态字"() -> (w352:refnum<vi>)
            n213 = case shown="0, 默认" w357 {
              tunnel: ["联网" ("connectionMode") "单机" ("connectionMode")] -> w358
              frame 1 {
              }
              frame 0, Default {
              }
            }
            "connectionMode" <- w358
            n214 = global write "Global.vi" "前序显示字"(w352) -> ()
            n215 = global write "Global.vi" "前序状态"(w353) -> ()
            "生产数量" <- w354
            "合格数量" <- w354
            "追溯码" <- "" ("输出轴码")
            "产品型号" <- "" ("productsName")
          }
          frame #1 {
            n216 = control-ref of="批次信息"() -> (w369:refnum<vi>)
            n217 = control-ref of="合格数量"() -> (w363:refnum<vi>)
            n218 = control-ref of="自动"() -> (w367:refnum<vi>)
            n219 = control-ref of="错误"() -> (w368:refnum<vi>)
            n220 = global write "Global.vi" "批次"(w369) -> ()
            n221 = global write "Global.vi" "合格数量"(w363) -> ()
            n222 = global write "Global.vi" "报警图标"(w368) -> ()
            n223 = global write "Global.vi" "程序自动"(w367) -> ()
            n224 = control-ref of="提示信息"() -> (w366:refnum<vi>)
            n225 = control-ref of="更换产品"() -> (w365:refnum<vi>)
            n226 = control-ref of="生产数量"() -> (w364:refnum<vi>)
            n227 = control-ref of="结果显示"() -> (w361:refnum<vi>)
            n228 = global write "Global.vi" "提示信息"(w366) -> ()
            n229 = control-ref of="检测结果"() -> (w362:refnum<vi>)
            n230 = global write "Global.vi" "生产数量"(w364) -> ()
            n231 = global write "Global.vi" "更换产品"(w365) -> ()
            n232 = global write "Global.vi" "检测结果"(w362) -> ()
            n233 = global write "Global.vi" "结果显示"(w361) -> ()
          }
          frame #2 {
            w370 = "" ("值")
            n234 = global read "Global.vi" "前序显示字"() -> (w372:refnum<vi>)
            n235 = global read "Global.vi" "前序状态"() -> (w371:refnum<vi>)
            n236 = vi-ref "A170316-11_config.vi"() -> (w383:refnum<vi>)
            n237 = call "浮动通知.vi"("通知内容"="请选择产品") -> ()  [unwired: 11 in]
            n238 = global read "Global.vi" "结果显示"() -> (w378:refnum<vi>)
            n239 = call "CallVI.vi"("VI引用"=w383, "状态"=T2."Standard") -> ()  [unwired: 11 in, 3 out]
            n240 = call "Colour.vi"("result"=w370, "colourRef"=w371) -> ()  [unwired: 9 in, 1 out]
            n241 = property class="Str"(reference=w372, "Value"=w370) -> ()  [unwired: 1 in, 2 out]
            n242 = property class="Str"(reference=w378, "Value"="..." ("结果显示")) -> (reference out=w381:refnum<vi>)  [unwired: 1 in, 1 out]
            n243 = property class="Str"(reference=w381, "Text.TextColor"=u32 16776960) -> ()  [unwired: 1 in, 2 out]
            n244 = call "看板状态.vi"("附加信息"="", "设备状态"=enum16{"设备离线", "设备正常", "设备缺料", "设备故障", "质量报警"}."设备正常") -> ("错误输出"=w373:errorcluster)  [unwired: 9 in]
            n245 = vi-ref "client.vi"() -> (w377:refnum<vi>)
            n246 = call "CallVI.vi"("VI引用"=w377, "状态"=T2."Hidden", "错误输入"=w373) -> ()  [unwired: 10 in, 3 out]
          }
        }
        n247 = call <vilib>:"Add State(s) to Queue__jki_lib_state_machine.vi"("State(s) in (\"\")"=w351) -> ("States Out"=w350:string)  [unwired: 14 in]
      }
      frame "UI: Cursor Set" {
        # "Argument"
        n248 = case shown="\"Idle\", 默认" w385 {
          tunnel: w387 -> [w392 w394]
          tunnel: [w391 w393] -> w386
          frame "Idle", Default {
            n249 = call <vilib>:"Unset Busy.vi"("error in (no error)"=w392) -> ("error out"=w391:errorcluster)  [unwired: 10 in]
          }
          frame "Busy" {
            n250 = call <vilib>:"Set Busy.vi"("error in (no error)"=w394) -> ("error out"=w393:errorcluster)  [unwired: 9 in, 1 out]
          }
        }
        n251 = call <vilib>:"Add State(s) to Queue__jki_lib_state_machine.vi"("State(s) in (\"\")"=w390) -> ("States Out"=w389:string)  [unwired: 14 in]
      }
      frame "UI: Front Panel State" {
        # "Argument"
        n252 = Unbundle By Name(w397) -> ("Core.Current VI Reference"=w396:refnum<vi>)
        n253 = case shown="\"Open\", 默认" w395 {
          tunnel: w399 -> [w405 w418]
          tunnel: [w407 w419] -> w398
          tunnel: w396 -> [w406 w416]
          frame "Open", Default {
            n254 = property class="VI"(reference=w406, error in=w405) -> (reference out=w403:refnum<vi>, error out=w404:errorcluster, "Front Panel.Open"=w402:bool)
            n255 = case shown="真" w402 {
              tunnel: [w410 w413] -> w407
              tunnel: w404 -> [w409 w413]
              tunnel: w403 -> [w408 _]
              frame False {
                n256 = invoke class="VI" method="FP.Open"(reference=w408, error in=w409, "Activate"=TRUE, "State"=T2."Standard") -> (error out=w410:errorcluster)  [unwired: 1 in, 4 out]
              }
              frame True {
              }
            }
          }
          frame "Close" {
            n257 = property class="VI"(reference=w416, error in=w418) -> (reference out=w415:refnum<vi>, error out=w417:errorcluster, "Front Panel.Open"=w414:bool)
            n258 = case shown="真" w414 {
              tunnel: [w420 w423] -> w419
              tunnel: w417 -> [w420 w422]
              tunnel: w415 -> [_ w421]
              frame False {
              }
              frame True {
                n259 = invoke class="VI" method="FP.Close"(reference=w421, error in=w422) -> (error out=w423:errorcluster)  [unwired: 1 in, 2 out]
              }
            }
          }
        }
        n260 = call <vilib>:"Add State(s) to Queue__jki_lib_state_machine.vi"("State(s) in (\"\")"=w401) -> ("States Out"=w400:string)  [unwired: 14 in]
      }
      frame "---------- Macro ----------" {
        n261 = call <vilib>:"Add State(s) to Queue__jki_lib_state_machine.vi"("State(s) in (\"\")"=w427) -> ("States Out"=w426:string)  [unwired: 14 in]
      }
      frame "Macro: Initialize" {
        w428 = "Data: Initialize\nInitialize Core Data\nS7: Initialize\nIdle\nUI: Initialize\nUI: Init\nUI: Front Panel State >> Open"  # Data: Initialize Initialize Core Data S7: Initialize Idle UI: Initialize UI: Init UI: Front Panel State >> Open
        n262 = call <vilib>:"Add State(s) to Queue__jki_lib_state_machine.vi"("State(s) in Front (\"\")"=w428, "State(s) in (\"\")"=w432) -> ("States Out"=w431:string)  [unwired: 13 in]
      }
      frame "Macro: Exit" {
        n263 = Unbundle By Name(w442) -> ("Core.Close Panel on Exit?"=w441:bool)
        n264 = vi-ref "client.vi"() -> (w435:refnum<vi>)
        n265 = invoke class="VI" method="FP.Close"(reference=w435) -> (reference out=w434:refnum<vi>, error out=w433:errorcluster)  [unwired: 2 in, 1 out]
        n266 = Close Reference(reference=w434, error in (no error)=w433) -> ()  [unwired: 1 out]
        n267 = Select(t="UI: Front Panel State >> Close", s=w441, f="") -> (s? t:f=w438:string)
        n268 = call <vilib>:"Add State(s) to Queue__jki_lib_state_machine.vi"("State(s) in (\"\")"=w438, "State(s) at Back (\"\")"="Data: Cleanup\nExit") -> ("States Out"=w436:string)  [unwired: 13 in]
        n269 = call <vilib>:"Add State(s) to Queue__jki_lib_state_machine.vi"("State(s) in Front (\"\")"=w436, "State(s) in (\"\")"=w445) -> ("States Out"=w444:string)  [unwired: 13 in]
      }
      frame "---------- New Category ----------" {
        n270 = call <vilib>:"Add State(s) to Queue__jki_lib_state_machine.vi"("State(s) in (\"\")"=w449) -> ("States Out"=w448:string)  [unwired: 14 in]
      }
      frame "New Category: 1" {
        n271 = call <vilib>:"Add State(s) to Queue__jki_lib_state_machine.vi"("State(s) in (\"\")"=w453) -> ("States Out"=w452:string)  [unwired: 14 in]
      }
      frame "New Category: 2" {
        n272 = call <vilib>:"Add State(s) to Queue__jki_lib_state_machine.vi"("State(s) in (\"\")"=w457) -> ("States Out"=w456:string)  [unwired: 14 in]
      }
    }
  }
